vi "ScanDelay_FTIR_BBnorm_Aligning.vi"() -> ()   [LabVIEW 2021] (continued)
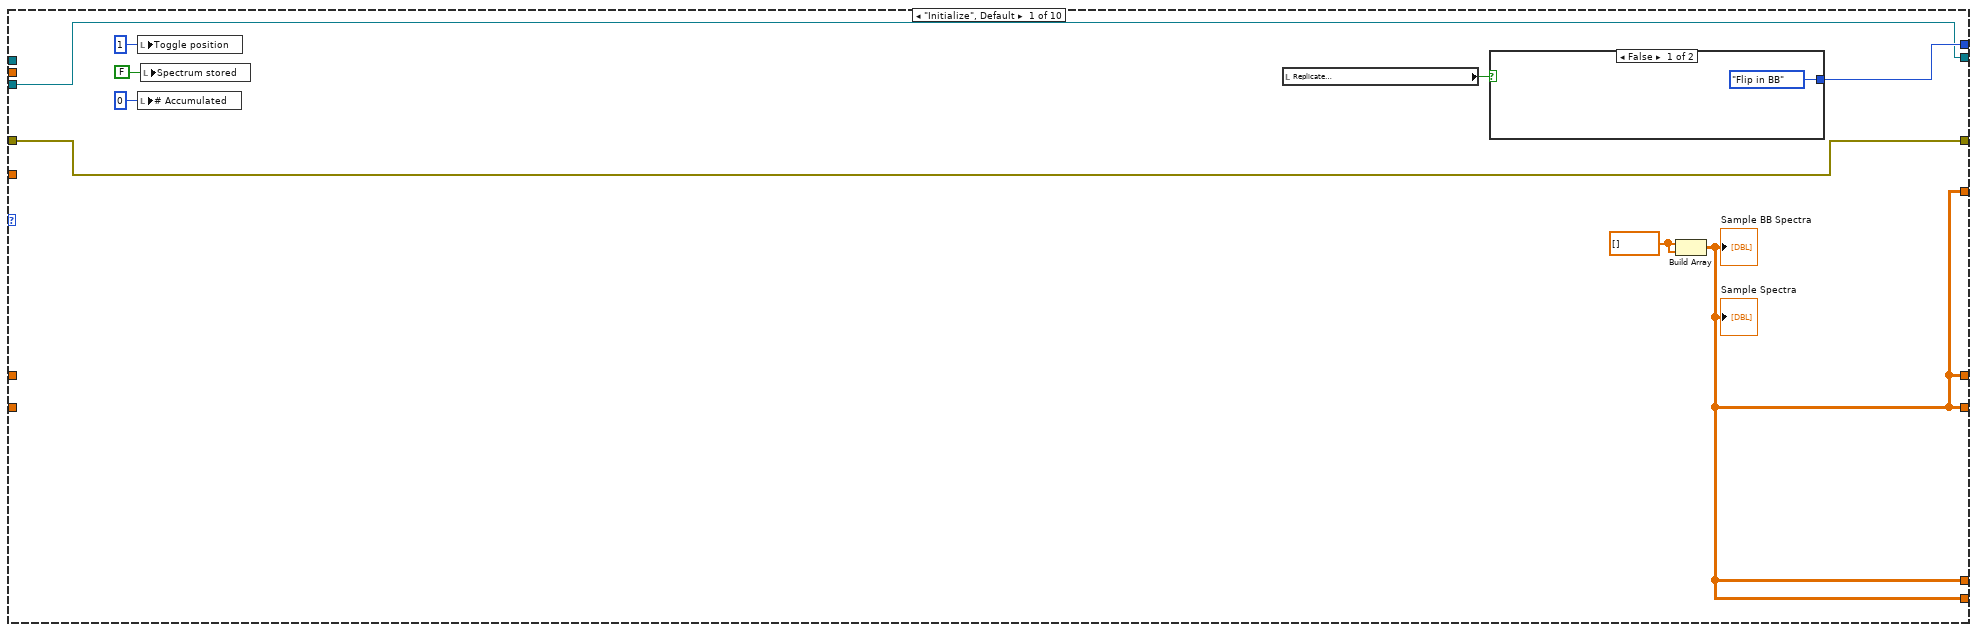
[diagram p3: hidden frame]
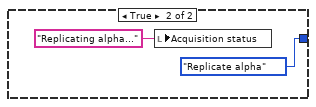
[diagram p4: hidden frame]
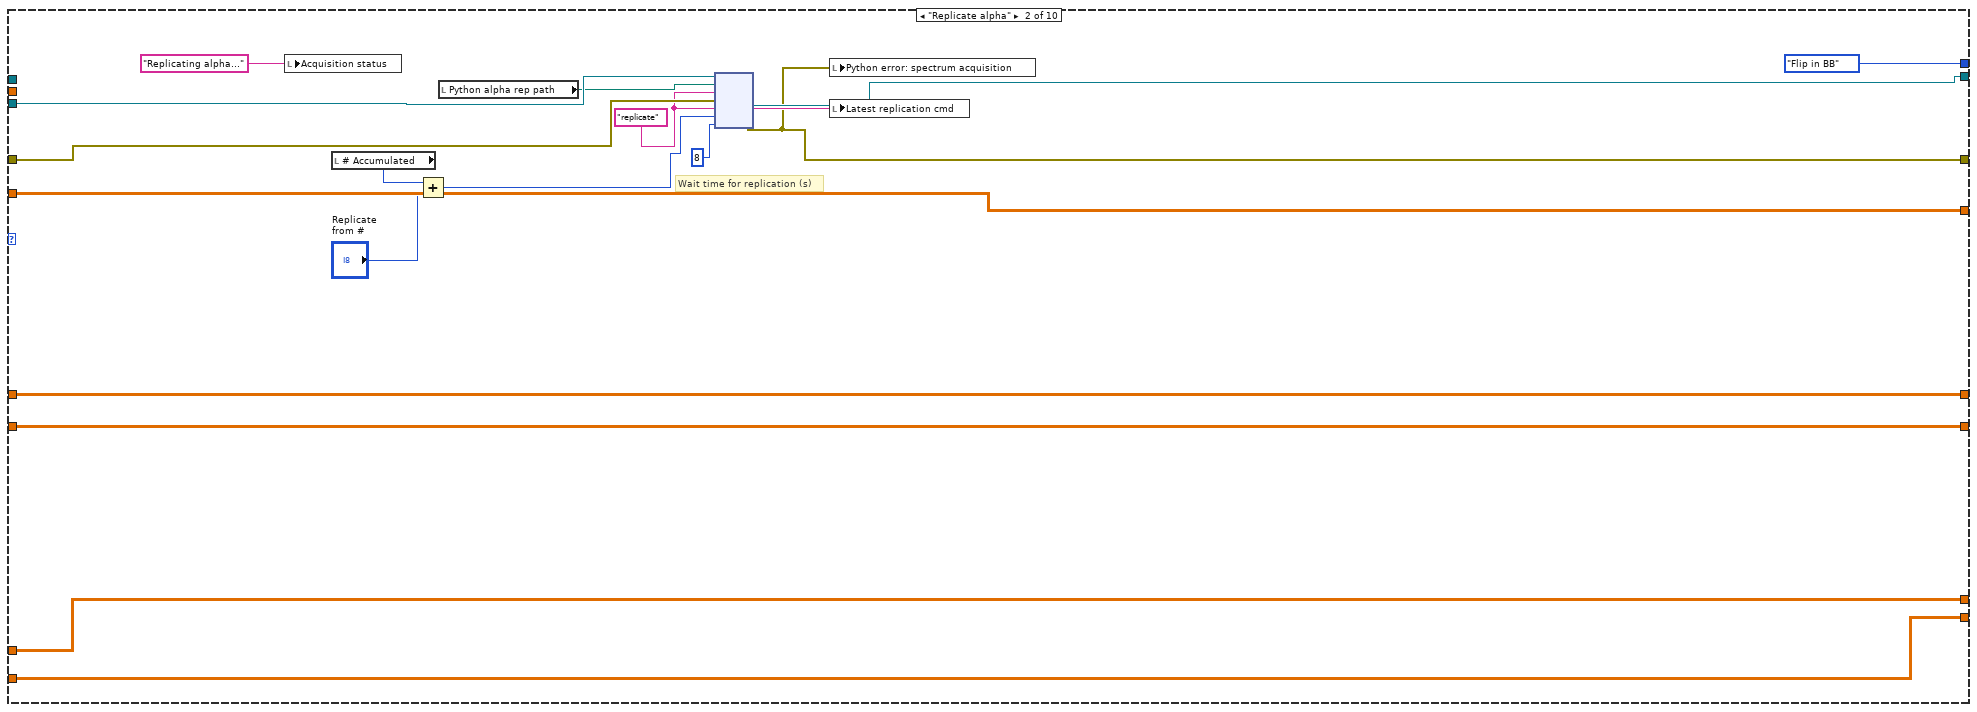
[diagram p5: hidden frame]
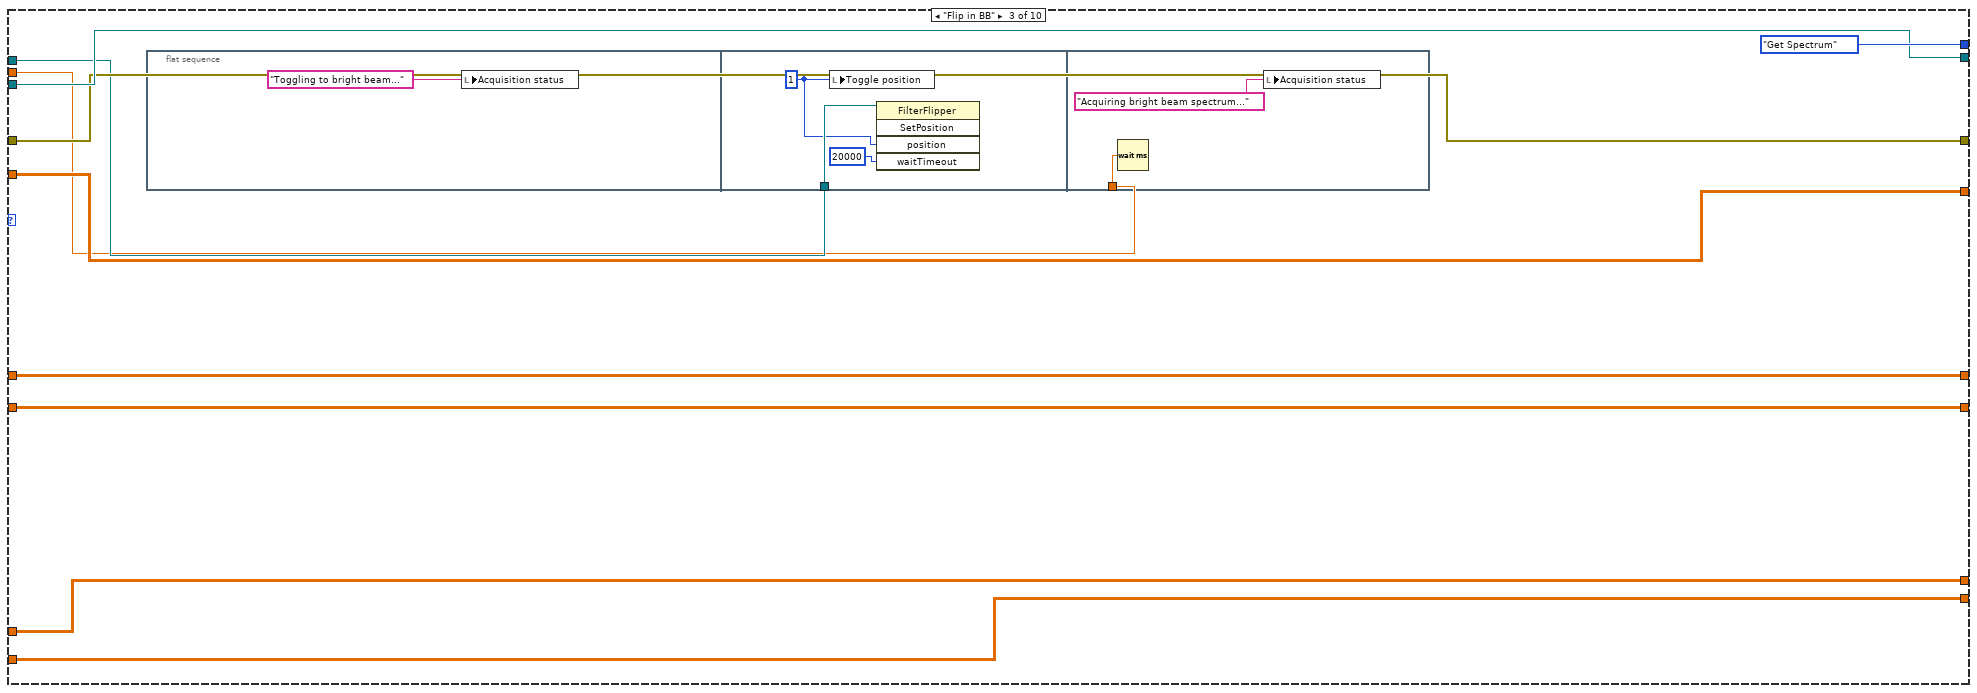
[diagram p6: hidden frame]
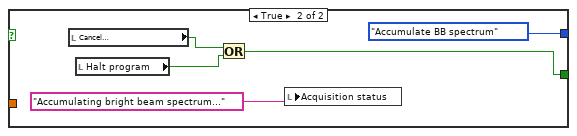
[diagram p8: hidden frame]
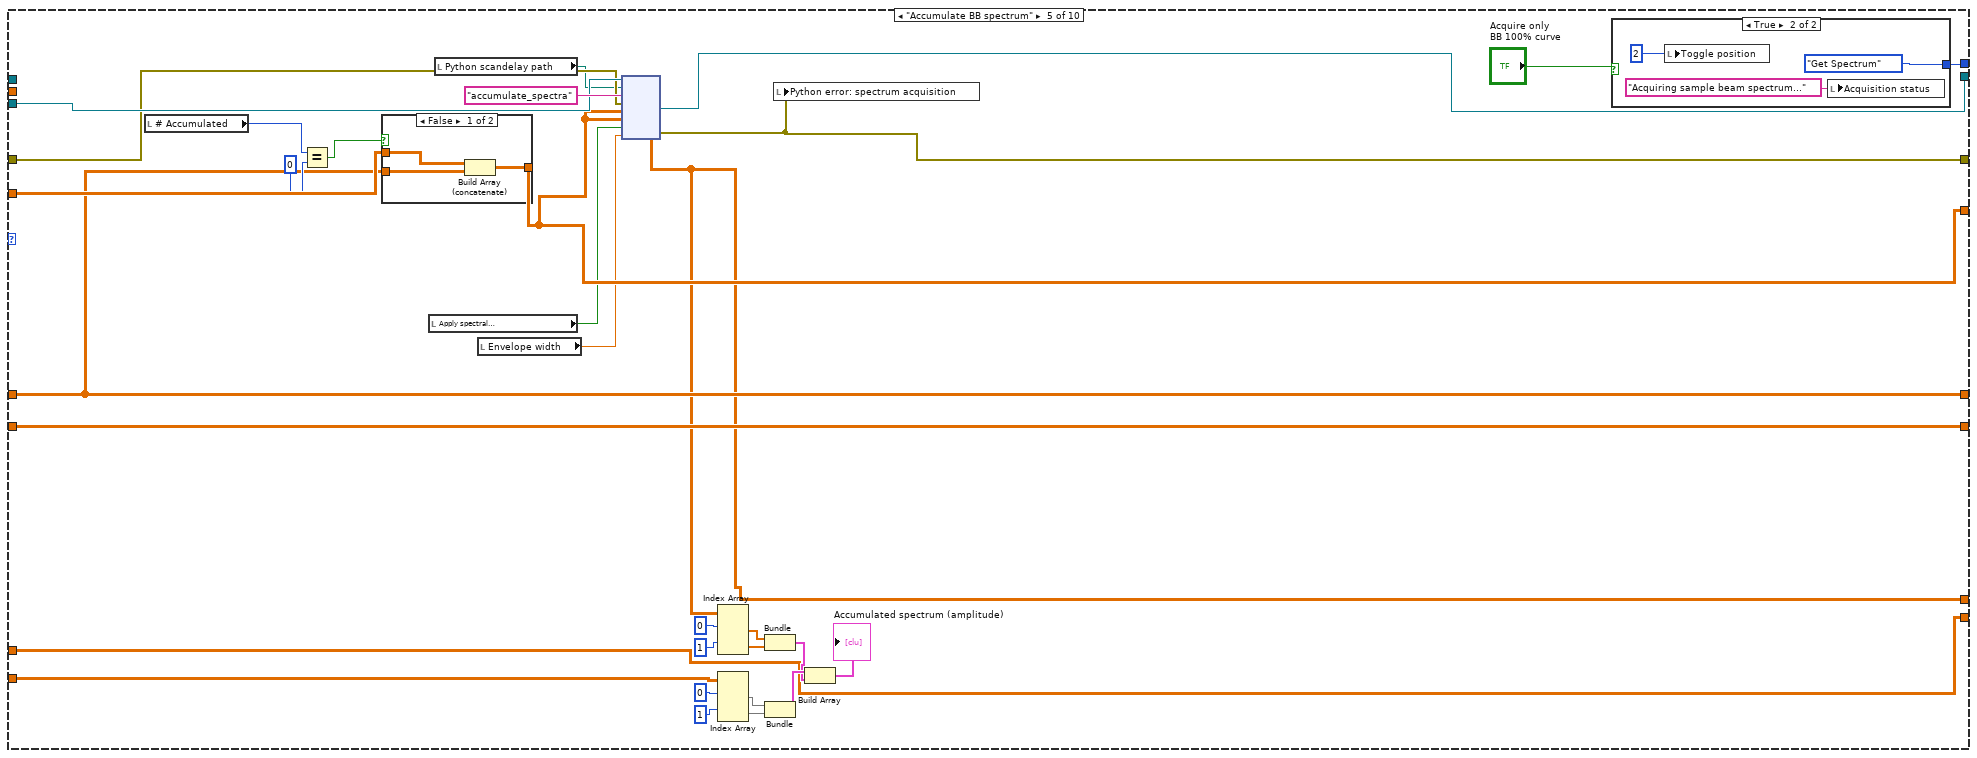
[diagram p9: hidden frame]
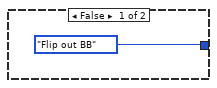
[diagram p10: hidden frame]
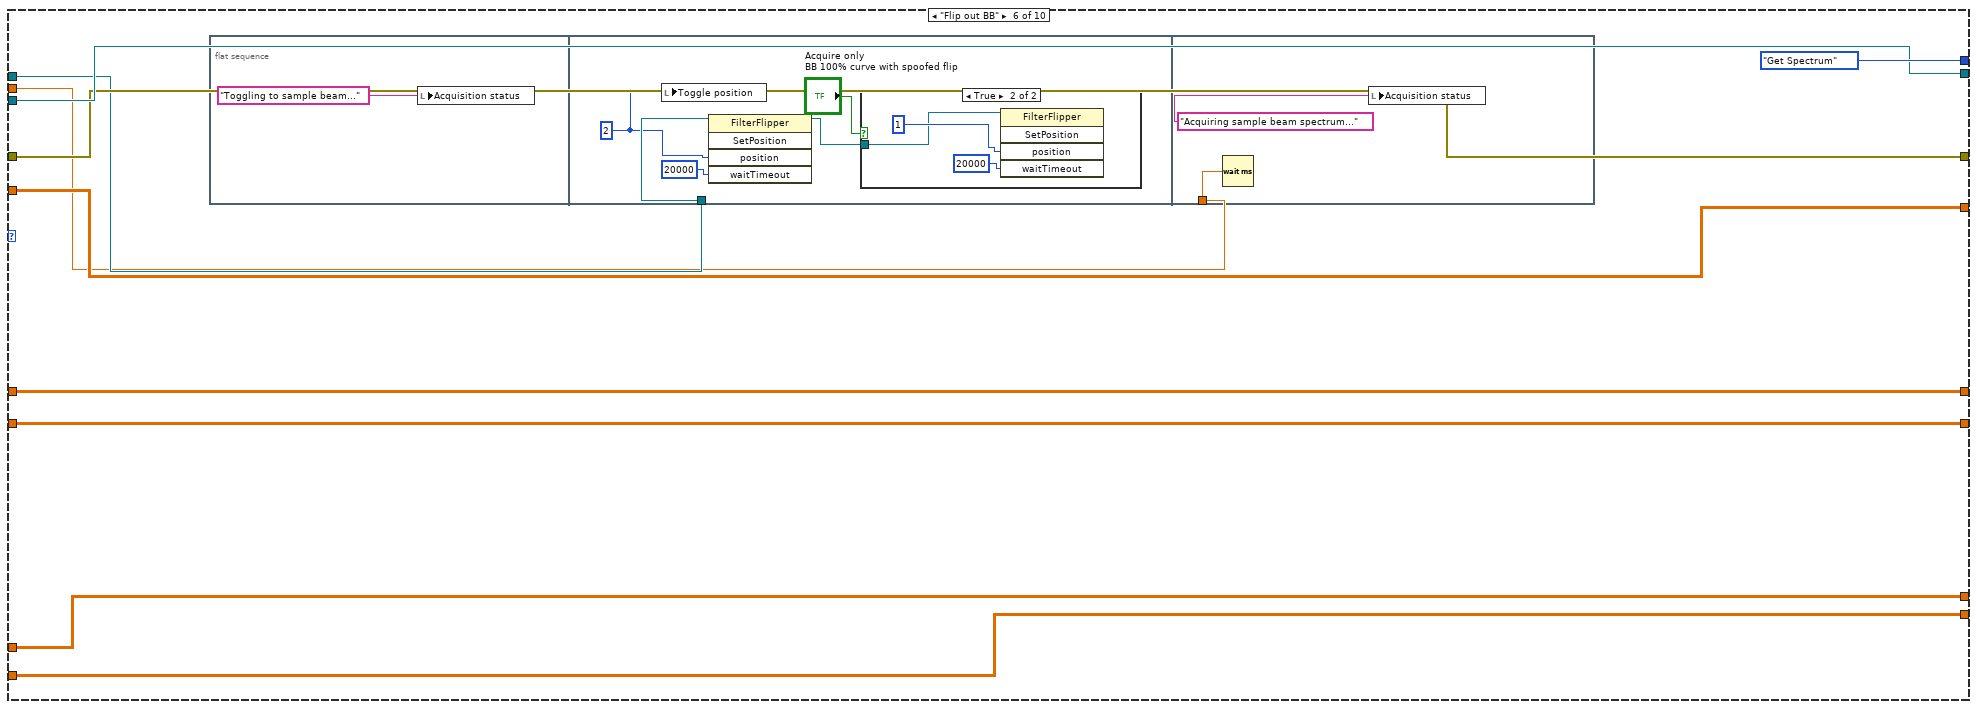
[diagram p12: hidden frame]
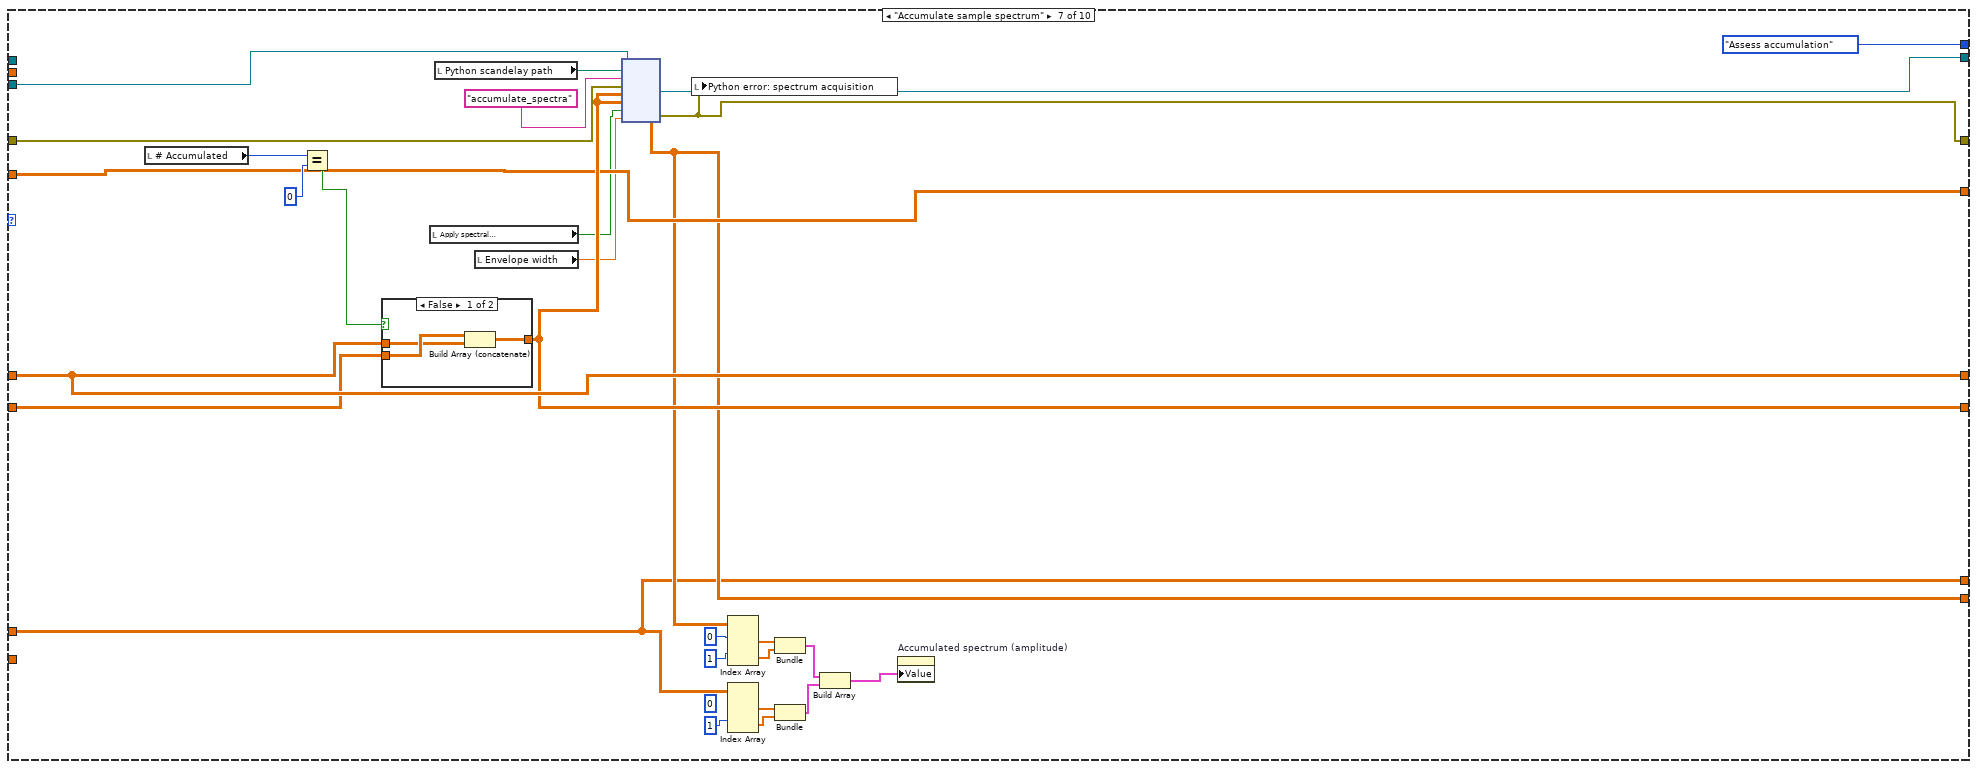
[diagram p14: hidden frame]
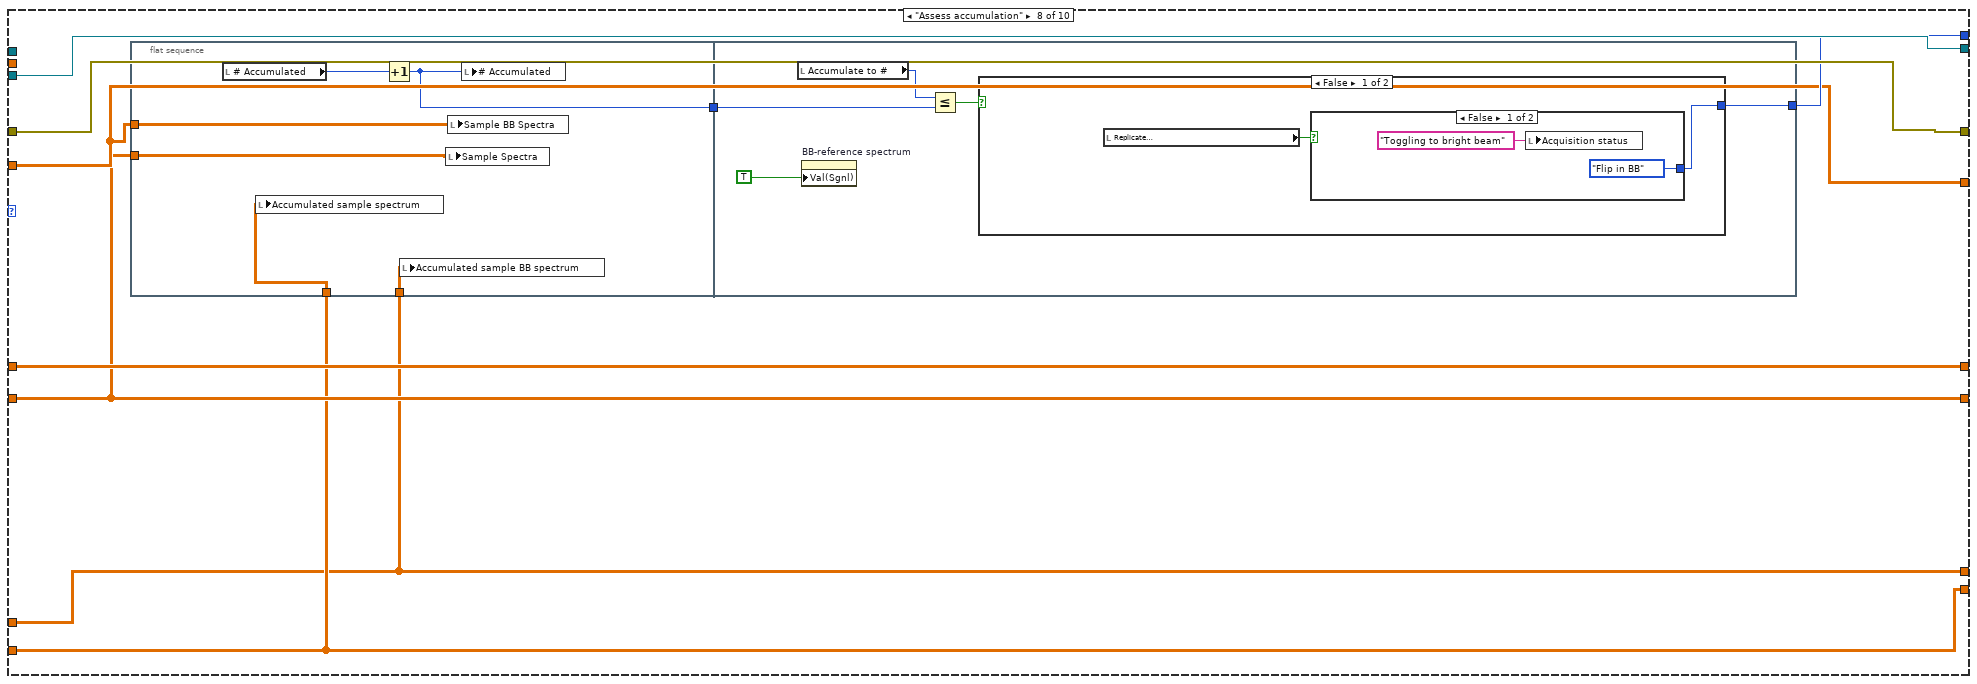
[diagram p16: hidden frame]
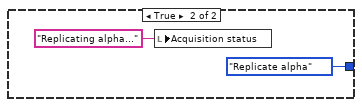
[diagram p17: hidden frame]
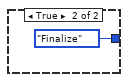
[diagram p18: hidden frame]
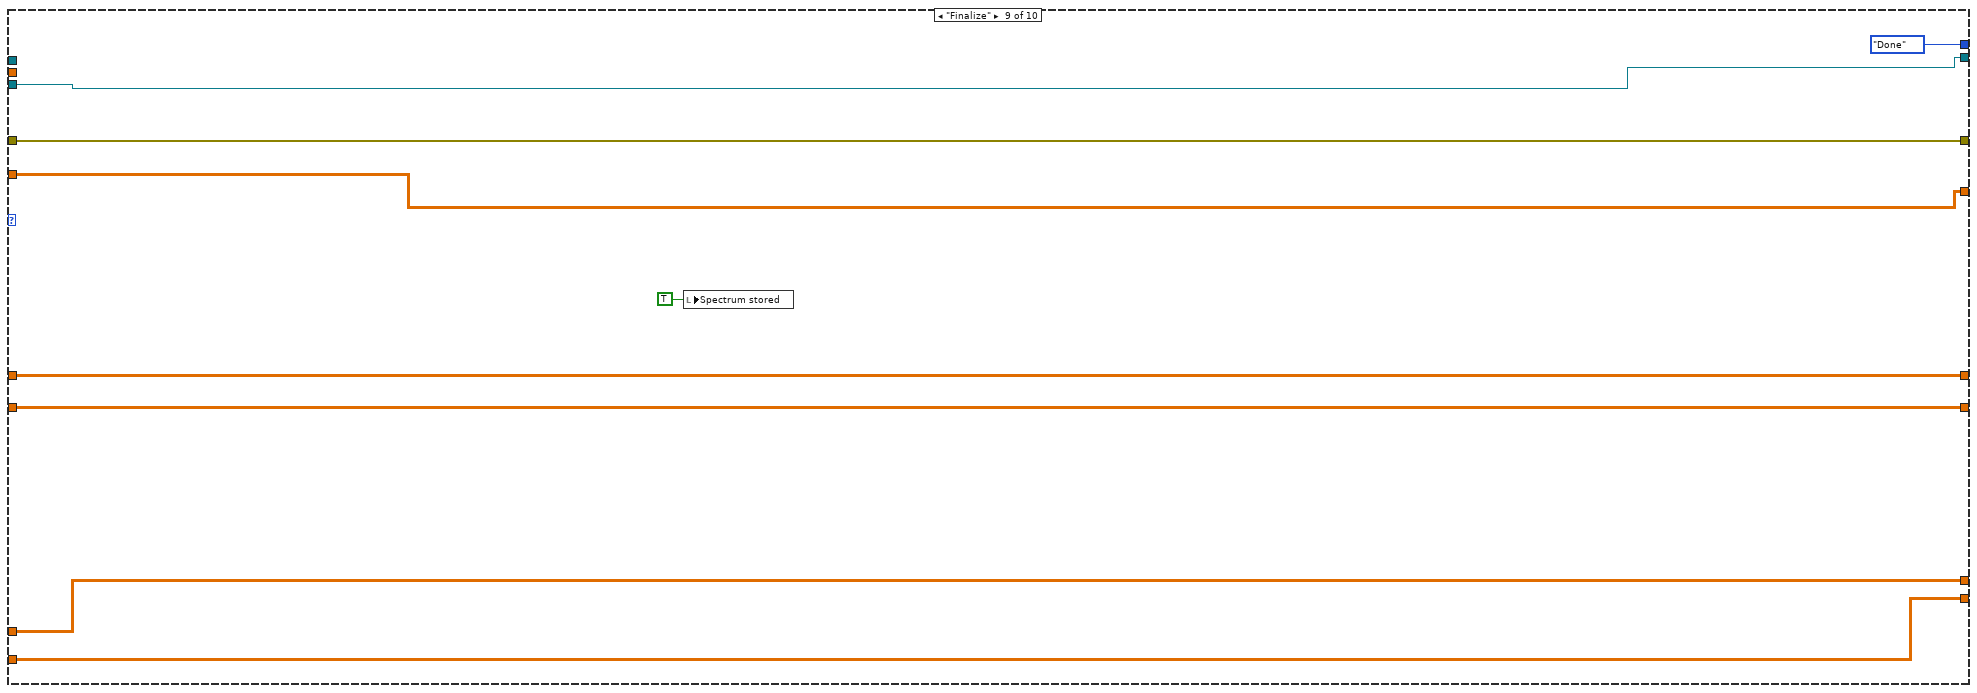
[diagram p19: hidden frame]
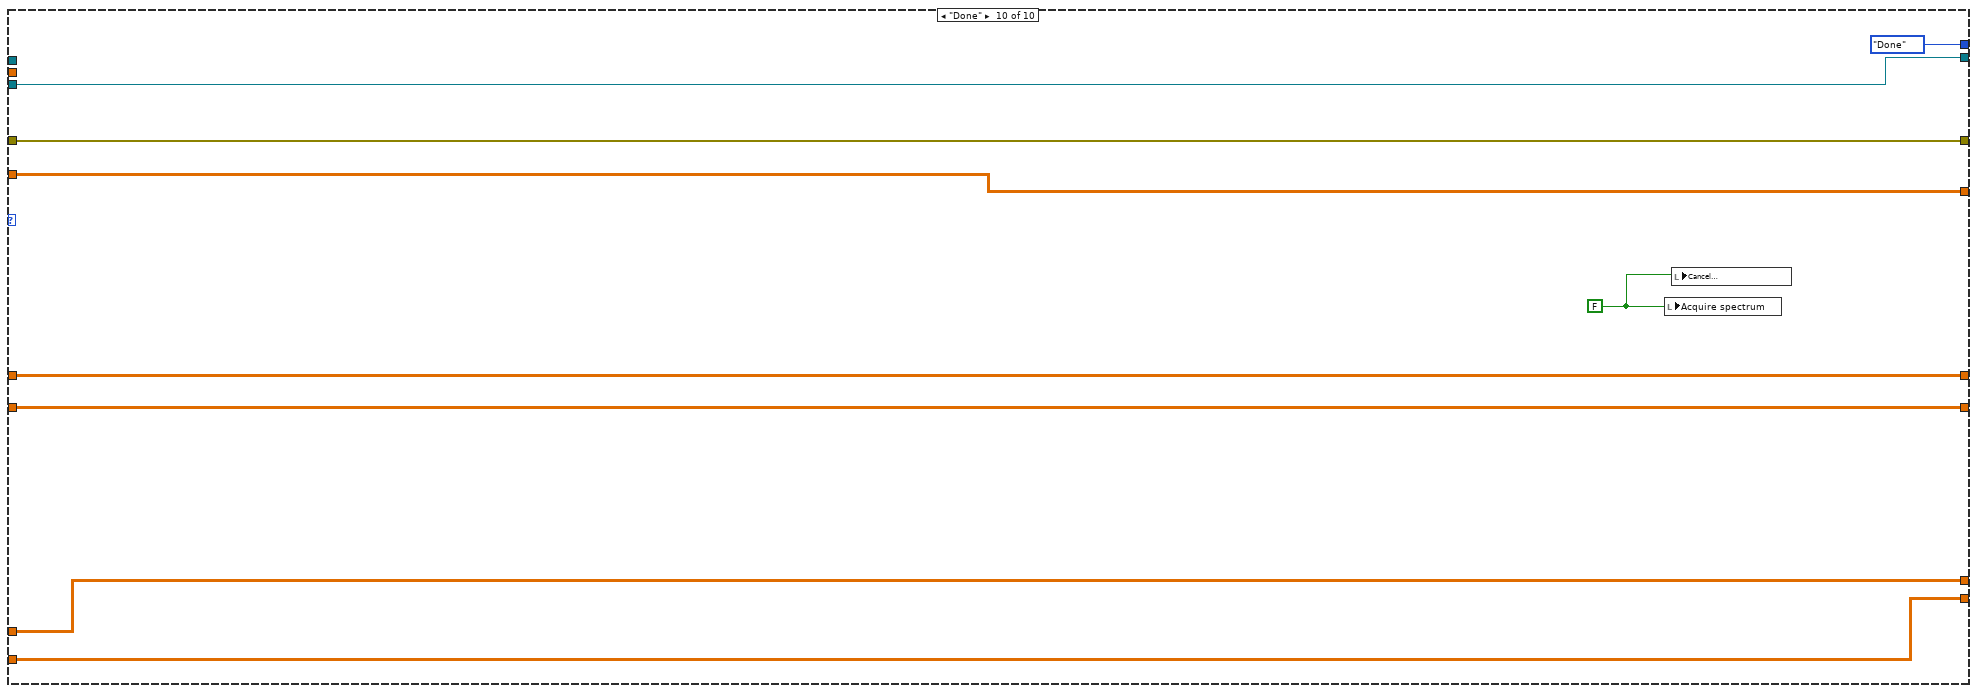
[diagram p20: hidden frame]
              n190 = Build Array(w368, w367) -> (→"Accumulated spectrum (amplitude)":T3)
              n191 = case shown="True" "Acquire only\nBB 100% curve" {
                tunnel: [Control_GetSpectrum_BBnorm."Flip out BB" Control_GetSpectrum_BBnorm."Get Spectrum"] -> w376
                frame False {
                }
                frame True {
                  n192 = local write "Toggle position"(2) -> ()
                  n193 = local write "Acquisition status"("Acquiring sample beam spectrum...") -> ()
                }
              }
            }
            frame "Flip out BB" {
              n194 = flat-sequence {
                tunnel: w403 -> [w415]
                tunnel: w402 -> [w419]
                frame #0 {
                  n195 = local write "Acquisition status"("Toggling to sample beam...") -> ()
                }
                frame #1 {
                  w413 = 2
                  n196 = local write "Toggle position"(w413) -> ()
                  n197 = invoke class="FilterFlipper" method="SetPosition"(reference=w415, "position"=w413, "waitTimeout"=20000) -> (reference out=w411:refnum<k24>)  [unwired: 2 in, 4 out]
                  n198 = case shown="True" "Acquire only\nBB 100% curve with spoofed flip" {
                    tunnel: w411 -> [_ w416]
                    frame False {
                    }
                    frame True {
                      n199 = invoke class="FilterFlipper" method="SetPosition"(reference=w416, "position"=1, "waitTimeout"=20000) -> ()  [unwired: 2 in, 5 out]
                    }
                  }
                }
                frame #2 {
                  n200 = Wait (ms)(milliseconds to wait=w419) -> ()  [unwired: 1 out]
                  n201 = local write "Acquisition status"("Acquiring sample beam spectrum...") -> ()
                }
              }
            }
            frame "Accumulate sample spectrum" {
              (unwired) 0
              n202 = local read "# Accumulated"() -> (w448:i32)
              n203 = Equal?(x=w448, y=0) -> (x = y?=w446:bool)
              n204 = case shown="False" w446 {
                tunnel: w436 -> [w450 w452]
                tunnel: w434 -> [w451 _]
                tunnel: [w449 w452] -> w433
                frame False {
                  n205 = Build Array (concatenate)(w451, w450) -> (w449:dbl[][])
                }
                frame True {
                }
              }
              n206 = local read "Apply spectral\nenvelope"() -> (w422:bool)
              n207 = local read "Python scandelay path"() -> (w441:path)
              n208 = local read "Envelope width"() -> (w421:dbl)
              n209 = node(w444, w441, "accumulate_spectra", w443, w433, w433, w422, w421) -> (w442:refnum<k35>, w432:errorcluster, w424:dbl[][])  [unwired: 3 in, 2 out]
              n210 = local write "Python error: spectrum acquisition"(w432) -> ()
              n211 = Index Array(array=w424, index (row) #1=0, index (row) #2=1) -> (element #1=w438:dbl[], element #2=w437:dbl[])  [unwired: 2 in]
              n212 = Index Array(array=w423, index (row) #2=1) -> (element #1=w429:dbl[], element #2=w428:dbl[])  [unwired: 3 in]
              n213 = Bundle("Output spectrum"=w438, "Output spectrum"=w437) -> (w431:T1)  [unwired: 1 in]
              n214 = Bundle("Output spectrum"=w429, "Output spectrum"=w428) -> (w427:T1)  [unwired: 1 in]
              n215 = Build Array(w431, w427) -> (w425:T3)
              n216 = property on="Accumulated spectrum (amplitude)" class="XYGraph (strict)"("Value"=w425) -> ()  [unwired: 2 in, 2 out]
            }
            frame "Assess accumulation" {
              n217 = flat-sequence {
                tunnel: [w466] -> w459
                tunnel: w456 -> [w465]
                tunnel: w455 -> [w464]
                tunnel: w454 -> [w462]
                tunnel: w453 -> [w463]
                tunnel: w459 -> [w468]
                tunnel: [w472] -> w458
                frame #0 {
                  n218 = local read "# Accumulated"() -> (w467:i32)
                  n219 = local write "Accumulated sample spectrum"(w462) -> ()
                  n220 = Increment(x=w467) -> (x+1=w466:i32)
                  n221 = local write "Accumulated sample BB spectrum"(w463) -> ()
                  n222 = local write "Sample Spectra"(w464) -> ()
                  n223 = local write "Sample BB Spectra"(w465) -> ()
                  n224 = local write "# Accumulated"(w466) -> ()
                }
                frame #1 {
                  n225 = local read "Accumulate to #"() -> (w469:i32)
                  n226 = property on="BB-reference spectrum" class="Bool (strict)"("Val(Sgnl)"=TRUE) -> ()  [unwired: 2 in, 2 out]
                  n227 = Less Or Equal?(x=w469, y=w468) -> (x <= y?=w470:bool)
                  n228 = case shown="False" w470 {
                    tunnel: [w473 Control_GetSpectrum_BBnorm."Finalize"] -> w472
                    frame False {
                      n229 = local read "Replicate\nalpha on\naccumulation"() -> (w474:bool)
                      n230 = case shown="False" w474 {
                        tunnel: [Control_GetSpectrum_BBnorm."Flip in BB" Control_GetSpectrum_BBnorm."Replicate alpha"] -> w473
                        frame False {
                          n231 = local write "Acquisition status"("Toggling to bright beam") -> ()
                        }
                        frame True {
                          n232 = local write "Acquisition status"("Replicating alpha...") -> ()
                        }
                      }
                    }
                    frame True {
                    }
                  }
                }
              }
            }
            frame "Finalize" {
              n233 = local write "Spectrum stored"(TRUE) -> ()
            }
            frame "Done" {
              w489 = FALSE
              n234 = local write "Acquire spectrum"(w489) -> ()
              n235 = local write "Cancel\nacquisition"(w489) -> ()
            }
          }
          n236 = Wait (ms)(milliseconds to wait=5) -> ()  [unwired: 1 out]
        }
      }
      event Timeout {
        n237 = event-data() -> ()  [unwired: 1 in, 3 out]
        n238 = Wait (ms)(milliseconds to wait=w500) -> ()  [unwired: 1 out]
      }
    }
    n239 = Wait (ms)(milliseconds to wait=5) -> ()  [unwired: 1 out]
    n240 = local read "Halt program"() -> (w243:bool)
    "Acquisition status" <- "Ready to acquire spectrum"
  }
  n241 = Close Python Session(session in=w18, error in=w17) -> (11:w14:errorcluster)
  n242 = local write "Python error: activity loop"(w14) -> ()
  n243 = Close Python Session(session in=w3, error in=w2) -> ()  [unwired: 1 out]
